vi "Nicolet 8.vi"(3 "?":u16(ring)=14 items=["16", "32", "64", "128", "256", "512", "1024", "2048", "4096", "8192", "16384", "32768", "65536", "131072", "262144", "524288 (one channel)", ""], 5 "Sample Duration (sec)":u32(knob)=29 scale=1.0..33.0) -> (0 "Waveform Graph":waveform(dbl)[](graph)=[{"t0"=timestamp(0 s since 1904-01-01), "dt"=0.00048828125, "Y"=array[133120 elements]}, {"t0"=timestamp(0 s since 1904-01-01), "dt"=0.00048828125, "Y"=array[133120 elements]}], 2 "data":dbl[][](array[numeric]) format="%0.2f", 8 "points":i32)   [LabVIEW 2010]
doc: "I. Description:\nThis example demonstrates how to acquire a finite amount of data (Waveform) using the DAQ device's internal clock, started by an analog edge condition.\n\nII. Instructions for Running:\n1. Select the physical channel to correspond to where your signal is input on the DAQ device.\n2. Enter the minimum and maximum voltage range.\nNote: For better accuracy try to match the input range to the expected voltage level of the measured signal.\n3. Set the number of samples to acquire per channel.\n4. Set the rate of the acquisition\nNote: The rate should be AT LEAST twice as fast as the maximum frequency component of the signal being acquired.\n5. Set the source of the start trigger. By default this is PFI0\n6. Set the slope and level of desired analog edge condition.\n\nIII. Block Diagram Steps:\n1. Create an empty task.\n2. Create an analog input voltage channel.\n3. Set the rate for the sample clock. Additionally, define the sample mode to be finite.\n4. Define the parameters for an Analog Slope Start Trigger.\n5. Call the Start VI to start the acquisition.\n6. Read all of the data.\n7. Stop the Analog Input Task.\n8. Call the Clear Task VI to clear the Task.\n9. Use the popup dialog box to display an error if any\nIV. I/O Connections Overview:\nMake sure your signal input terminal matches the Physical Channel I/O Control. In this case wire your signal to the ai0 pin on your DAQ Device."
uses:
  Detection/200262.llb/Trigger Select.ctl
  <vilib>/Utility/error.llb/DialogType.ctl
  <vilib>/DAQmx/write.llb/DAQmx Write (Analog DBL 1Chan 1Samp).vi
  <vilib>/DAQmx/read.llb/DAQmx Read (Analog 2D DBL NChan NSamp).vi
  <vilib>/DAQmx/create/channels.llb/DAQmx Create Channel (AO-Voltage-Basic).vi
  <vilib>/daqmx/miscellaneous.llb/DAQmx Fill In Error Info.vi
  <vilib>/DAQmx/create/channels.llb/DAQmx Create Channel (AI-Voltage-Basic).vi
  <vilib>/DAQmx/configure/timing.llb/DAQmx Timing (Sample Clock).vi
  <vilib>/DAQmx/configure/trigger.llb/DAQmx Start Trigger (Analog Edge).vi
  <vilib>/DAQmx/configure/trigger.llb/DAQmx Reference Trigger (Digital Edge).vi
  <vilib>/measure/maspectr.llb/FFT Power Spectral Density for 1 Chan.vi
  <vilib>/measure/NI_MAPro.lvlib
panel:
  in  "Sample Rate Hz":bool
  out "Cursor Time Selected":dbl=0.07992895204262879
  out "Cursor Peak to Peak Voltage":dbl=11.550802139037433
  in  "File Name":path=path "signalaverage.lvm"
  in  "Save Average To File":bool
  out "Pretrigger Samples":dbl=6656.0
  out "Seconds Per Division":dbl=0.1
  out "Posttrigger Samples Captured":dbl=133120.0
  in  "Voltage Offset":dbl(knob) scale=-2.0..2.0
  in  "Average / Live Display":bool=TRUE
  in  "Seconds  Per Division":u32(knob) min=1 max=1 step=1 scale=0.0..15.0
  out "Samples Averaged":i32
  in  "Averaging Enabled":bool
  in  "Volts Per Division":dbl(knob)=1.0 scale=0.005..5.0
  in  "Pretrigger Duration (%)":dbl(knob)=0.05 min=0.0 max=2.0 step=1.0 scale=0.05..0.95
  in  "Analog Source":string="Dev1/ai30"
  in  "Digital External TTL Source":tag="/Dev1/PFI0"
  in  "Trigger Type":T1
  in  "Analog Edge Level":dbl format="%0.2f"
  in  "Edge":i32(ring)=10280 items=["Rising"=10280, "Falling"=10171]
  in  "Physical Channel":tag="Dev1/ai23, Dev1/ai22" caption="Physical Channels"
  out "Sampling Iterations":i32
  in  "Maximum  Voltage":dbl=10.0
  in  "Minimum Voltage":dbl=-10.0
  out "Sampling Rate":i32=2048 caption="Sample Rate (Hz)"
  in  "stop":bool=TRUE
  # "Channel\nConfiguration"
  # "Triggering Parameters"
  # "Voltage Parameters"
  # "TTL Trigger Options"
  # "Timing Parameters"
  # "External  Trigger Options"
  # "Storage Options"
  # "Nicolet 8.vi*If X scale markers are not drawn:\nRight click the waveform diagram -> select X axis -> marker spacing -> set to arbitrary AFTER\nsetting the correct seconds per division"
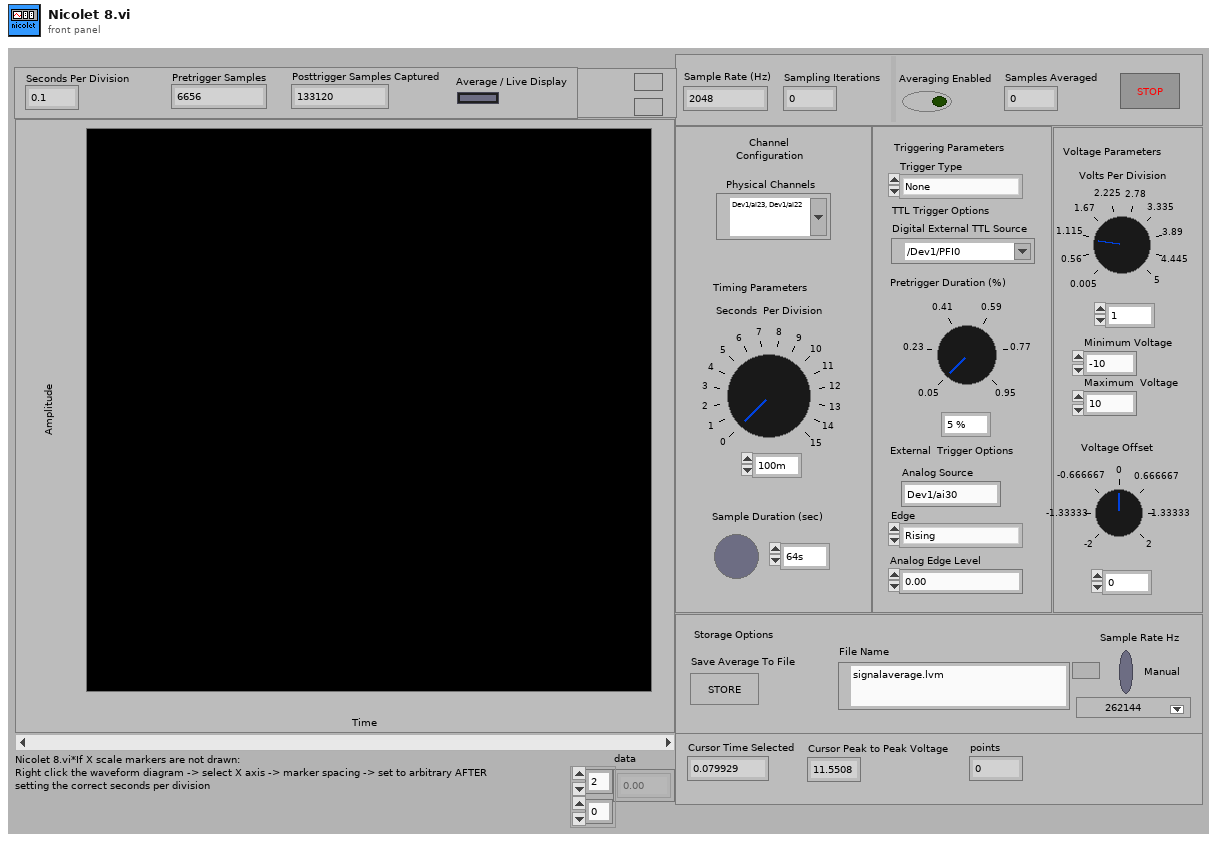
[diagram p1: front panel]
types:
  T1 = typedef "Trigger Select.ctl" = enum16{"None", "Analog Edge", "Digital Edge"}
  T2 = typedef "DialogType.ctl" = u16
  T3 = typedef "LVCursorListTypeDef.ctl" = cluster{"Name":string, "Color":u32, "Style":u8, "Point Style":u8, "Name Visible":bool, "Allow Drag":bool, "Cursor Mode":u32, "Plot":i32, "Index":i32, "Position":cluster{"X":dbl, "Y":dbl}, "X Scale":u32, "Y Scale":u32, "Watch Plots":i32[], "Watch All Plots":bool, "Plot Area":i32, "Label Offset":cluster{"X":dbl, "Y":dbl}}[]
  T4 = cluster{"Name":string, "Color":u32, "Style":u8, "Point Style":u8, "Name Visible":bool, "Allow Drag":bool, "Cursor Mode":u32, "Plot":i32, "Index":i32, "Position":cluster{"X":dbl, "Y":dbl}, "X Scale":u32, "Y Scale":u32, "Watch Plots":i32[], "Watch All Plots":bool, "Plot Area":i32, "Label Offset":cluster{"X":dbl, "Y":dbl}}
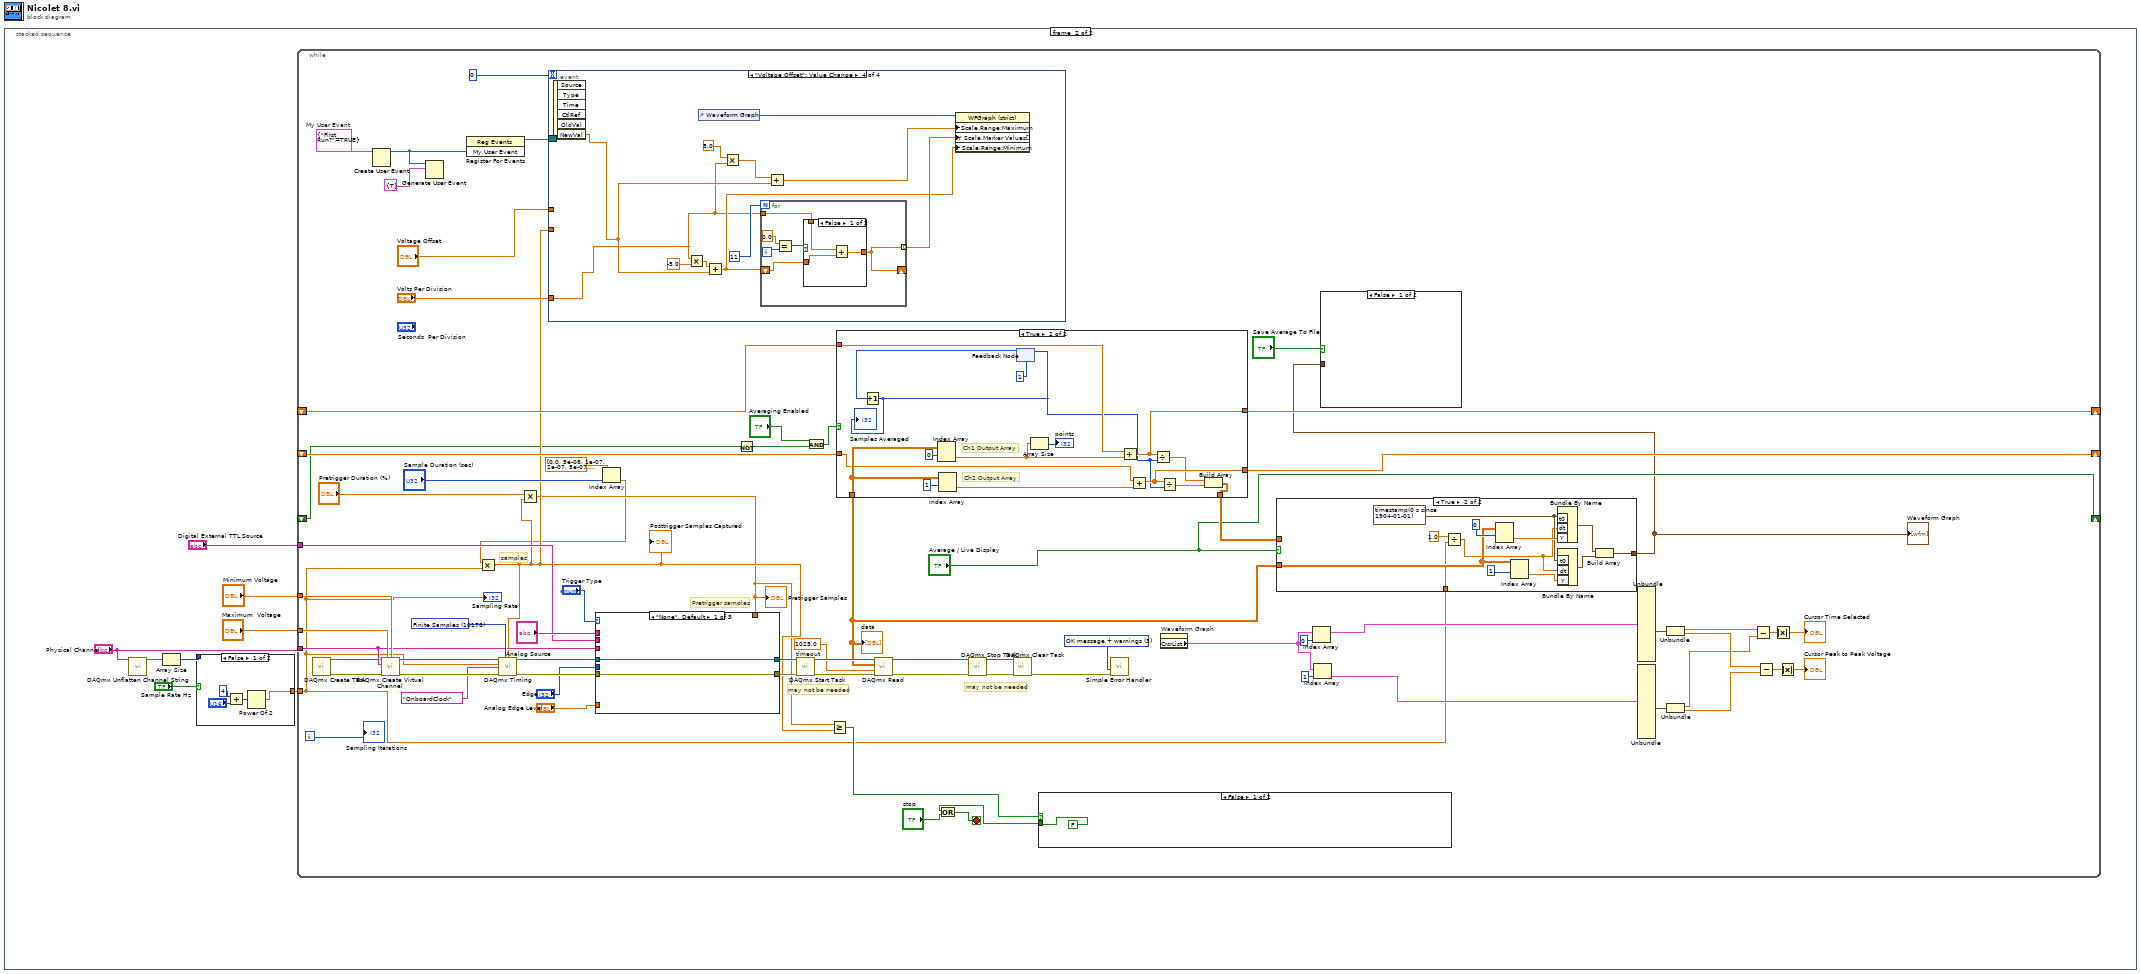
[diagram p0: block diagram]
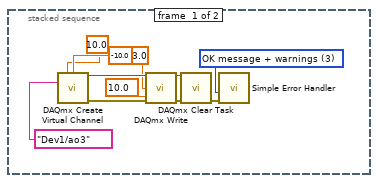
[diagram p2: hidden frame]
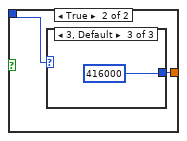
[diagram p3: hidden frame]
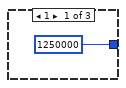
[diagram p4: hidden frame]
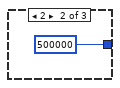
[diagram p5: hidden frame]
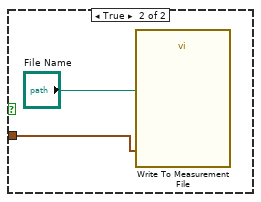
[diagram p6: hidden frame]
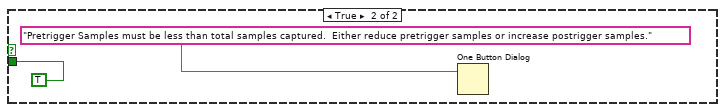
[diagram p7: hidden frame]
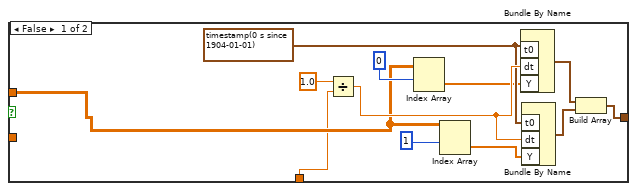
[diagram p8: hidden frame]
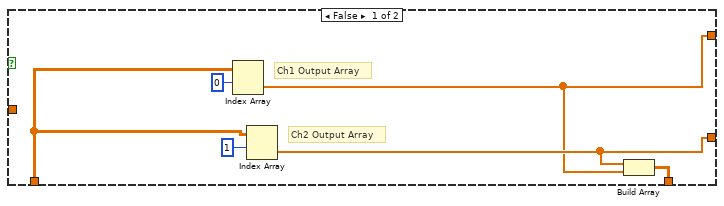
[diagram p9: hidden frame]
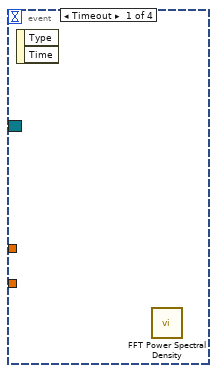
[diagram p10: hidden frame]
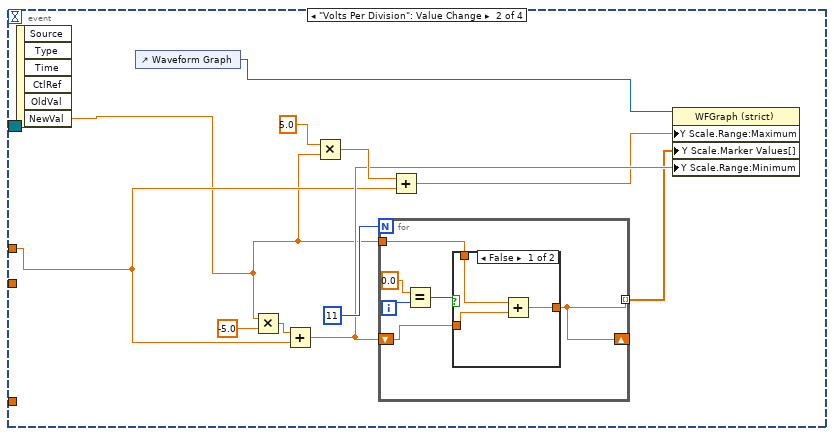
[diagram p11: hidden frame]
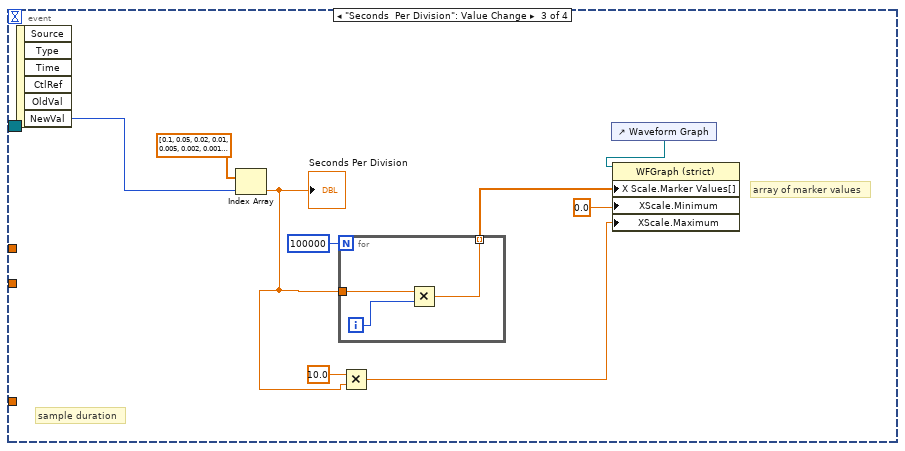
[diagram p13: hidden frame]
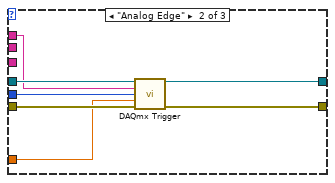
[diagram p15: hidden frame]
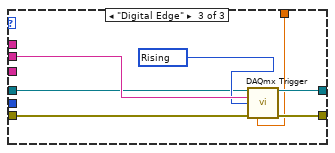
[diagram p16: hidden frame]
diagram:
  n1 = stacked-sequence {
    frame #0 {
      w4 = T2 3 items=["no dialog", "OK message", "continue or stop message", "OK message + warnings", "continue/stop + warnings"] ("type of dialog (OK msg:1)")
      n2 = call-poly <vilib>:"DAQmx Create Virtual Channel.vi"("maximum value"=10.0 ("Maximum Value"), "minimum value"=-10.0 ("Minimum Value"), "physical channels"=tag "Dev1/ao3" ("Physical Channel")) -> ("task out"=w7:refnum<k21>, "error out"=w8:errorcluster)  [unwired: 6 in, 5 out]
      n3 = call-poly <vilib>:"DAQmx Write.vi"("task/channels in"=w7, "data"=3.0 ("Voltage Output"), "timeout"=10.0, "error in"=w8) -> ("task out"=w2:refnum<k21>, "error out"=w3:errorcluster)  [unwired: 1 in, 9 out]
      n4 = call <vilib>:"DAQmx Clear Task.vi"("task in"=w2, "error in"=w3) -> ("error out"=w1:errorcluster)  [unwired: 13 out]
      n5 = call <vilib>:"Simple Error Handler.vi"("type of dialog (OK msg:1)"=w4, "error in (no error)"=w1) -> ()  [unwired: 8 out]
    }
    frame #1 {
      n6 = call <vilib>:"DAQmx Unflatten Channel String.vi"("names in"="Physical Channel") -> ("names out"=w15:string[])  [unwired: 1 in, 13 out]
      n7 = Array Size(array=w15) -> (size(s)=w13:i32)
      n8 = case shown="False" "Sample Rate Hz" {
        tunnel: [w21 w25] -> w14
        tunnel: w13 -> [_ w24]
        frame False {
          n9 = Add(x=4, y="?") -> (x+y=w22:i32)
          n10 = Power Of 2(x=w22) -> (2^x=w21:dbl)
        }
        frame True {
          n11 = case shown="3, Default" w24 {
            tunnel: [1250000 500000 416000] -> w25
            frame 1 {
            }
            frame 2 {
            }
            frame 3, Default {
            }
          }
        }
      }
      n12 = while {
        tunnel: "Minimum Voltage" -> [w82]
        tunnel: "Maximum  Voltage" -> [w81]
        tunnel: "Physical Channel" -> [w80]
        tunnel: "Digital External TTL Source" -> [w78]
        shift-right: [w72] -> _
        shift-left: _ -> [w71]
        shift-right: [w66] -> _
        shift-left: _ -> [w65]
        tunnel: w14 -> [w33]
        shift-right: ["Average / Live Display"] -> _
        shift-left: _ -> [w36]
        i -> [w92]
        stop <- w58 stop-if-true
        w77 = cluster{"First Run?":bool} {"First Run?"=TRUE}  # My User Event
        w98 = T2 3 items=["no dialog", "OK message", "continue or stop message", "OK message + warnings", "continue/stop + warnings"] ("type of dialog (OK msg:1)")
        w95 = 1025.0  # timeout
        w93 = 10178 items=["Finite Samples"=10178, "Continuous Samples"=10123] ("sample mode")
        # "samples"
        # "may not be needed"
        # "may not be needed"
        # "Pretrigger samples"
        n13 = call <vilib>:"DAQmx Create Task.vi"() -> ("task out"=w69:refnum<k21>, "error out"=w68:errorcluster)  [unwired: 5 in, 9 out]
        n14 = Create User Event(user event datatype=w77) -> (user event=w75:refnum<user-event>)  [unwired: 1 in, 1 out]
        n15 = call-poly <vilib>:"DAQmx Create Virtual Channel.vi"("task in"=w69, "maximum value"=w81, "minimum value"=w82, "physical channels"=w80, "error in"=w68) -> ("task out"=w94:refnum<k21>, "error out"=w102:errorcluster)  [unwired: 4 in, 5 out]
        n16 = Generate User Event(user event=w75, event data cluster=cluster{"First Run?":bool} {"First Run?"=TRUE} ("event data")) -> ()  [unwired: 1 in, 2 out]
        n17 = register-events(w75) -> (reference out=w73:refnum<event-registration>)  [unwired: 2 in, 1 out]
        n18 = Index Array(array=dbl[] [0.0, 5e-08, 1e-07, 2e-07, 5e-07, 1e-06, 2e-06, 5e-06, 1e-05, 2e-05, 5e-05, 0.0001, 0.0002, 0.0005, 0.001, 0.002, 0.005, 0.01, 0.02, 0.05, 0.1, 0.2, 0.5, 1.0, 2.0, 5.0, 10.0, 16.5, 32.5, 65.0, 129.0, 257.0, 513.0, 1025.0], index="Sample Duration (sec)") -> (element=w32:dbl)
        n19 = Multiply(x=w32, y=w33) -> (x*y=w56:dbl)
        "Posttrigger Samples Captured" <- w56
        n20 = call-poly <vilib>:"DAQmx Timing.vi"("task/channels in"=w94, "sample mode"=w93, "samples per channel"=w56, "rate"=w33, "source"=tag "OnboardClock", "error in"=w102) -> ("task out"=w87:refnum<k21>, "error out"=w85:errorcluster)  [unwired: 1 in, 7 out]
        n21 = Multiply(x="Pretrigger Duration (%)", y=w56) -> (x*y=w55:dbl)
        "Pretrigger Samples" <- w55
        n22 = event shown="[3] \"Voltage Offset\": Value Change" {
          selector: w73 -> [_ _ _ _]
          dyn-events: _ -> [_ _ _ _]
          timeout: 0 -> [_ _ _ _]
          tunnel: w56 -> [_ _ _ _]
          tunnel: "Voltage Offset" -> [_ w156 _ _]
          tunnel: "Volts Per Division" -> [_ _ _ w188]
          event Timeout {
            n23 = event-data() -> ()  [unwired: 3 out]
            n24 = call-poly <vilib>:"FFT Power Spectral Density.vi"() -> ()  [unwired: 6 in, 6 out]
          }
          event "Volts Per Division": Value Change {
            n25 = event-data() -> ("NewVal"=w155:dbl)  [unwired: 6 out]
            n26 = control-ref of="Waveform Graph"() -> (w154:refnum<vi>)
            n27 = Multiply(x=w155, y=-5.0) -> (x*y=w161:dbl)
            n28 = Add(x=w161, y=w156) -> (x+y=w159:dbl)
            n29 = Multiply(x=5.0, y=w155) -> (x*y=w160:dbl)
            n30 = for {
              N: 11 -> [_]
              tunnel: w155 -> [w170]
              tunnel: [w169] -> w157 mode=indexing
              shift-right: [w169] -> _
              shift-left: w159 -> [w167]
              i -> [w165]
              n31 = Equal?(x=0.0, y=w165) -> (x = y?=w168:bool)
              n32 = case shown="False" w168 {
                tunnel: w170 -> [w173 _]
                tunnel: w167 -> [w172 w174]
                tunnel: [w171 w174] -> w169
                frame False {
                  n33 = Add(x=w173, y=w172) -> (x+y=w171:dbl)
                }
                frame True {
                }
              }
            }
            n34 = Add(x=w160, y=w156) -> (x+y=w158:dbl)
            n35 = property on="Property Node" class="WFGraph (strict)"(reference=w154, "Y Scale.Range:Maximum"=w158, "Y Scale.Marker Values[]"=w157, "Y Scale.Range:Minimum"=w159) -> ()  [unwired: 1 in, 2 out]
          }
          event "Seconds  Per Division": Value Change {
            # "sample duration"
            # "array of marker values"
            n36 = event-data() -> ("NewVal"=w182:u32)  [unwired: 6 out]
            n37 = Index Array(array=dbl[] [0.1, 0.05, 0.02, 0.01, 0.005, 0.002, 0.001, 0.0005, 0.0002, 0.0001, 5e-05, 2e-05, 1e-05, 5e-06, 2e-06, 1e-06], index=w182) -> (element=w176:dbl)
            "Seconds Per Division" <- w176
            n38 = for {
              N: 100000 -> [_]
              tunnel: w176 -> [w185]
              tunnel: [w184] -> w178 mode=indexing
              i -> [w186]
              n39 = Multiply(x=w185, y=w186) -> (x*y=w184:dbl)
            }
            n40 = Multiply(x=10.0, y=w176) -> (x*y=w175:dbl)
            n41 = control-ref of="Waveform Graph"() -> (w180:refnum<vi>)
            n42 = property on="Property Node" class="WFGraph (strict)"(reference=w180, "X Scale.Marker Values[]"=w178, "XScale.Minimum"=0.0 ("x"), "XScale.Maximum"=w175) -> ()  [unwired: 1 in, 2 out]
          }
          event "Voltage Offset": Value Change {
            n43 = event-data() -> ("NewVal"=w189:dbl)  [unwired: 6 out]
            n44 = Multiply(x=w188, y=-5.0) -> (x*y=w196:dbl)
            n45 = control-ref of="Waveform Graph"() -> (w187:refnum<vi>)
            n46 = Add(x=w196, y=w189) -> (x+y=w190:dbl)
            n47 = Multiply(x=5.0, y=w188) -> (x*y=w197:dbl)
            n48 = for {
              N: 11 -> [_]
              tunnel: w188 -> [w203]
              tunnel: [w202] -> w191 mode=indexing
              shift-right: [w202] -> _
              shift-left: w190 -> [w200]
              i -> [w198]
              n49 = Equal?(x=0.0, y=w198) -> (x = y?=w201:bool)
              n50 = case shown="False" w201 {
                tunnel: w203 -> [w206 _]
                tunnel: w200 -> [w205 w207]
                tunnel: [w204 w207] -> w202
                frame False {
                  n51 = Add(x=w206, y=w205) -> (x+y=w204:dbl)
                }
                frame True {
                }
              }
            }
            n52 = Add(x=w197, y=w189) -> (x+y=w192:dbl)
            n53 = property on="Property Node" class="WFGraph (strict)"(reference=w187, "Y Scale.Range:Maximum"=w192, "Y Scale.Marker Values[]"=w191, "Y Scale.Range:Minimum"=w190) -> ()  [unwired: 1 in, 2 out]
          }
        }
        n54 = case shown="\"None\", Default" "Trigger Type" {
          tunnel: w87 -> [w209 w212 w219]
          tunnel: [w209 w214 w223] -> w86
          tunnel: w85 -> [w208 w216 w218]
          tunnel: [w208 w213 w222] -> w84
          tunnel: w80 -> [_ _ _]
          tunnel: "Analog Edge Level" -> [_ w215 _]
          tunnel: "Analog Source" -> [_ w211 _]
          tunnel: w78 -> [_ _ w221]
          tunnel: w55 -> [_ _ w217]
          tunnel: "Edge" -> [_ w210 _]
          frame "None", Default {
          }
          frame "Analog Edge" {
            n55 = call-poly <vilib>:"DAQmx Trigger.vi"("task/channels in"=w212, "source"=w211, "slope"=w210, "level"=w215, "error in"=w216) -> ("task out"=w214:refnum<k21>, "error out"=w213:errorcluster)  [unwired: 9 out]
          }
          frame "Digital Edge" {
            w220 = 10280 items=["Rising"=10280, "Falling"=10171] ("edge")
            n56 = call-poly <vilib>:"DAQmx Trigger.vi"("task/channels in"=w219, "source"=w221, "edge"=w220, "error in"=w218, "pretrigger samples per channel"=w217) -> ("task out"=w223:refnum<k21>, "error out"=w222:errorcluster)  [unwired: 9 out]
          }
        }
        n57 = Not(x=w36) -> (.not. x?=w35:bool)
        n58 = call <vilib>:"DAQmx Start Task.vi"("task/channels in"=w86, "error in"=w84) -> ("task out"=w96:refnum<k21>, "error out"=w101:errorcluster)  [unwired: 12 out]
        n59 = And(x="Averaging Enabled", y=w35) -> (x .and. y?=w34:bool)
        n60 = Greater Or Equal?(x=w55, y=w56) -> (x >= y?=w60:bool)
        n61 = call-poly <vilib>:"DAQmx Read.vi"("task/channels in"=w96, "timeout"=w95, "error in"=w101) -> ("task out"=w91:refnum<k21>, "data"=w29:dbl[][], "error out"=w90:errorcluster)  [unwired: 1 in, 9 out]
        "data" <- w29
        n62 = case shown="True" w34 {
          tunnel: w29 -> [w135 w153]
          tunnel: [w133 w148] -> w72
          tunnel: w71 -> [_ w146]
          tunnel: [w134 w145] -> w66
          tunnel: w65 -> [_ w144]
          tunnel: [w132 w140] -> w53
          frame False {
            # "Ch2 Output Array"
            # "Ch1 Output Array"
            n63 = Index Array(array=w135, index (row)=0 ("disabled index (col)")) -> (element=w133:dbl[])  [unwired: 1 in]
            n64 = Index Array(array=w135, index (row)=1 ("disabled index (col)")) -> (element=w134:dbl[])  [unwired: 1 in]
            n65 = Build Array(w134, w133) -> (w132:dbl[][])
          }
          frame True {
            # "Ch2 Output Array"
            # "Ch1 Output Array"
            n66 = Index Array(array=w153, index (row)=0 ("disabled index (col)")) -> (element=w139:dbl[])  [unwired: 1 in]
            n67 = Index Array(array=w153, index (row)=1 ("disabled index (col)")) -> (element=w147:dbl[])  [unwired: 1 in]
            n68 = feedback #1(1) -> (w149:i32)
            n69 = Increment(x=w149) -> (x+1=w143:i32)
            "Samples Averaged" <- w143
            n70 = feedback-in #1(w143) -> ()
            n71 = Array Size(array=w139) -> (size(s)=→"points":i32)
            n72 = Add(x=w146, y=w139) -> (x+y=w148:dbl[])
            n73 = Add(x=w144, y=w147) -> (x+y=w145:dbl[])
            n74 = Divide(x=w148, y=w143) -> (x/y=w142:dbl[])
            n75 = Divide(x=w145, y=w143) -> (x/y=w141:dbl[])
            n76 = Build Array(w142, w141) -> (w140:dbl[][])
          }
        }
        n77 = call <vilib>:"DAQmx Stop Task.vi"("task/channels in"=w91, "error in"=w90) -> ("task out"=w97:refnum<k21>, "error out"=w100:errorcluster)  [unwired: 12 out]
        n78 = call <vilib>:"DAQmx Clear Task.vi"("task in"=w97, "error in"=w100) -> ("error out"=w99:errorcluster)  [unwired: 13 out]
        n79 = case shown="False" w60 {
          tunnel: [FALSE TRUE] -> w57
          frame False {
          }
          frame True {
            n80 = One Button Dialog(message="Pretrigger Samples must be less than total samples captured.  Either reduce pretrigger samples or increase postrigger samples.") -> ()  [unwired: 2 out]
          }
        }
        n81 = Or(x=w57, y="stop") -> (x .or. y?=w58:bool)
        n82 = call <vilib>:"Simple Error Handler.vi"("type of dialog (OK msg:1)"=w98, "error in (no error)"=w99) -> ()  [unwired: 8 out]
        n83 = property on="Waveform Graph" class="WFGraph (strict)"() -> ("CrsrList"=w31:T3)  [unwired: 2 in, 2 out]
        n84 = case shown="True" "Average / Live Display" {
          tunnel: w29 -> [_ w128]
          tunnel: [w110 w120] -> w30
          tunnel: w53 -> [w112 _]
          tunnel: w33 -> [w111 w124]
          frame False {
            w117 = timestamp(0 s since 1904-01-01) ("t0")
            n85 = Divide(x=1.0, y=w111) -> (x/y=w119:dbl)
            n86 = Index Array(array=w112, index (row)=0 ("disabled index (col)")) -> (element=w113:dbl[])  [unwired: 1 in]
            n87 = Index Array(array=w112, index (row)=1 ("disabled index (col)")) -> (element=w116:dbl[])  [unwired: 1 in]
            n88 = Bundle By Name("t0"=w117, "dt"=w119, "Y"=w113) -> (w108:waveform(dbl))  [unwired: 1 out]
            n89 = Bundle By Name("t0"=w117, "dt"=w119, "Y"=w116) -> (w109:waveform(dbl))  [unwired: 1 out]
            n90 = Build Array(w108, w109) -> (w110:waveform(dbl)[])
          }
          frame True {
            w126 = timestamp(0 s since 1904-01-01) ("t0")
            n91 = Divide(x=1.0, y=w124) -> (x/y=w123:dbl)
            n92 = Index Array(array=w128, index (row)=0 ("disabled index (col)")) -> (element=w131:dbl[])  [unwired: 1 in]
            n93 = Index Array(array=w128, index (row)=1 ("disabled index (col)")) -> (element=w127:dbl[])  [unwired: 1 in]
            n94 = Bundle By Name("t0"=w126, "dt"=w123, "Y"=w131) -> (w121:waveform(dbl))  [unwired: 1 out]
            n95 = Bundle By Name("t0"=w126, "dt"=w123, "Y"=w127) -> (w122:waveform(dbl))  [unwired: 1 out]
            n96 = Build Array(w121, w122) -> (w120:waveform(dbl)[])
          }
        }
        "Waveform Graph" <- w30
        n97 = Index Array(array=w31, index=0) -> (element=w50:T4)
        n98 = Index Array(array=w31, index=1) -> (element=w49:T4)
        n99 = case shown="False" "Save Average To File" {
          tunnel: w30 -> [_ w103]
          frame False {
          }
          frame True {
            n100 = call "Write To Measurement File"("Signals"=w103, "File Name"="File Name") -> ()  [unwired: 5 in, 13 out]
          }
        }
        n101 = Unbundle(w50) -> ("Position"=w48:cluster{"X":dbl, "Y":dbl})  [unwired: 15 out]
        n102 = Unbundle(w49) -> ("Position"=w47:cluster{"X":dbl, "Y":dbl})  [unwired: 15 out]
        n103 = Unbundle(w48) -> ("X"=w42:dbl, "Y"=w46:dbl)
        n104 = Unbundle(w47) -> ("X"=w40:dbl, "Y"=w45:dbl)
        n105 = Subtract(x=w42, y=w40) -> (x-y=w41:dbl)
        n106 = Subtract(x=w46, y=w45) -> (x-y=w44:dbl)
        n107 = Absolute Value(x=w41) -> (abs(x)=→"Cursor Time Selected":dbl)
        n108 = Absolute Value(x=w44) -> (abs(x)=→"Cursor Peak to Peak Voltage":dbl)
        "Sampling Rate" <- w33
        "Sampling Iterations" <- w92
      }
    }
  }
